vi "Laser Ablation and Capture.vi"() -> ()   [LabVIEW 2016] (continued)
          }
          frame True {
          }
        }
      }
    }
    n235 = call "uc480_SubVI_Example_SyncEventLoop.vi"("Error In"=w84, "use sync"=w86, ".NET (Reference)"=w85) -> ("Error Out"=w82:errorcluster, "Synchronize (ms)"=w83:dbl)  [unwired: 7 in]
    "Error Out" <- w82
    n236 = Wait Until Next ms Multiple(millisecond multiple=w83) -> ()  [unwired: 1 out]
  }
  n237 = flat-sequence "Initialization sequence" {
    tunnel: [w597] -> w38
    tunnel: [w581] -> w36
    tunnel: [w580] -> w35
    tunnel: [w577] -> w33
    tunnel: [w576] -> w32
    tunnel: [w573] -> w21
    tunnel: [w572] -> w2
    tunnel: [w571] -> w1
    tunnel: w38 -> [w739]
    tunnel: [w733] -> w37
    tunnel: w36 -> [w732]
    tunnel: w35 -> [w731]
    tunnel: [w730] -> w34
    tunnel: w33 -> [w730]
    tunnel: w32 -> [w729]
    tunnel: [w729] -> w31
    tunnel: [w728] -> w22
    tunnel: w21 -> [w728]
    tunnel: [w727] -> w10
    tunnel: [w726] -> w6
    tunnel: w2 -> [w727]
    tunnel: w1 -> [w726]
    tunnel: [w754] -> w49
    tunnel: [w745] -> w48
    tunnel: [w746] -> w44
    tunnel: w37 -> [w750]
    tunnel: w34 -> [w744]
    tunnel: w31 -> [w743]
    tunnel: [w742] -> w23
    tunnel: w22 -> [w742]
    tunnel: w10 -> [w741]
    tunnel: [w741] -> w9
    tunnel: w6 -> [w740]
    tunnel: [w740] -> w5
    tunnel: w49 -> [w760]
    tunnel: [w760] -> w47
    tunnel: w48 -> [w759]
    tunnel: [w758] -> w45
    tunnel: w44 -> [w758]
    tunnel: [w757] -> w30
    tunnel: w23 -> [w757]
    tunnel: w9 -> [w756]
    tunnel: [w756] -> w8
    tunnel: w5 -> [w755]
    tunnel: [w755] -> w4
    tunnel: w47 -> [w767]
    tunnel: [w767] -> w46
    tunnel: w45 -> [w766]
    tunnel: w30 -> [w765]
    tunnel: [w765] -> w29
    tunnel: w8 -> [w764]
    tunnel: [w764] -> w7
    tunnel: w4 -> [w763]
    tunnel: [w763] -> w3
    tunnel: [w777] -> w43
    tunnel: w46 -> [w777]
    tunnel: w29 -> [w772]
    tunnel: [w772] -> w28
    tunnel: [w771] -> w20
    tunnel: [w770] -> w15
    tunnel: w7 -> [w771]
    tunnel: w3 -> [w770]
    tunnel: w43 -> [w782]
    tunnel: [w782] -> w42
    tunnel: w28 -> [w780]
    tunnel: [w780] -> w27
    tunnel: w20 -> [w779]
    tunnel: [w779] -> w19
    tunnel: w15 -> [w778]
    tunnel: [w778] -> w14
    tunnel: w42 -> [w787]
    tunnel: [w787] -> w41
    tunnel: w27 -> [w785]
    tunnel: [w785] -> w26
    tunnel: w19 -> [w784]
    tunnel: [w784] -> w18
    tunnel: w14 -> [w783]
    tunnel: [w783] -> w13
    tunnel: w41 -> [w792]
    tunnel: [w792] -> w40
    tunnel: w26 -> [w790]
    tunnel: [w790] -> w25
    tunnel: w18 -> [w789]
    tunnel: [w789] -> w17
    tunnel: w13 -> [w788]
    tunnel: [w788] -> w12
    tunnel: w40 -> [w797]
    tunnel: [w797] -> w39
    tunnel: w25 -> [w795]
    tunnel: [w795] -> w24
    tunnel: w17 -> [w794]
    tunnel: [w794] -> w16
    tunnel: w12 -> [w793]
    tunnel: [w793] -> w11
    tunnel: w39 -> [w801]
    tunnel: w24 -> [w800]
    tunnel: w16 -> [w799]
    tunnel: w11 -> [w798]
    frame #0 {
      w598 = "standby" ("regular expression")
      w608 = FALSE ("Visible")
      n238 = control-ref of="This VI"() -> (w609:refnum<vi>)
      n239 = control-ref of="This VI"() -> (w607:refnum<vi>)
      n240 = invoke class="VI" method="Default Vals.Reinit All"(reference=w609) -> ()  [unwired: 2 in, 3 out]
      n241 = property on="Axes Manual Control" class="Bool (strict)"("Visible"=w608) -> ()  [unwired: 2 in, 2 out]
      n242 = property on="Home Axes" class="Bool"("Visible"=w608) -> ()  [unwired: 2 in, 2 out]
      n243 = property class="VI"(reference=w607) -> ("Path"=w606:path)  [unwired: 1 in, 2 out]
      n244 = Strip Path(path=w606) -> (stripped path=w605:path)  [unwired: 1 out]
      n245 = Build Path(base path=w605, name or relative path="General_Configuration.ini") -> (appended path=w603:path)
      n246 = call <vilib>:"Open Config Data.vi"("create file if necessary (T)"=FALSE, "configuration file path"=w603) -> ("error out"=w578:errorcluster, "refnum"=w579:T5)  [unwired: 7 in, 1 out]
      n247 = call "Configuration reader.vi"("refnum"=w579, "error in (no error)"=w578) -> ("Velocity"=→"Velocity":dbl, "Exposure"=w572:dbl, "X offset"=w590:i32, "Y travel"=w588:dbl, "X travel"=w587:dbl, "Y offset"=w589:i32, "Acceleration"=→"Acceleration":dbl, "Pixelclock"=w573:i32, "Framerate"=w571:dbl, "Width (px)"=w592:i32, "Speed (µm/s)"=w596:i32, "XPS_Address"=→"XPS_Address":string, "Axis 1 group"=w577:i32, "Precision (%)"=w593:dbl, "Pixel size"=w594:dbl, "Axis 2 inverted?"=→"Axis 2 inverted?":bool, "Axis 1 inverted?"=→"Axis 1 inverted?":bool, "Heigth (px)"=w591:i32, "Laser Com Delay"=w580:i32, "Height  step \ndivider"=w595:i32, "VISA Laser port"=w581:string, "Axis 2 group"=w576:i32, "error out"=w583:errorcluster)  [unwired: 3 in]
      "VISA Laser port" <- w581
      "Laser Com Delay" <- w580
      "Axis 1 group" <- w577
      "Axis 2 group" <- w576
      n248 = local write "Heigth (px)"(w591) -> ()
      n249 = local write "Pixel size"(w594) -> ()
      n250 = local write "Precision (%)"(w593) -> ()
      n251 = local write "Speed (µm/s)"(w596) -> ()
      n252 = local write "Width (px)"(w592) -> ()
      n253 = local write "Y offset"(w590) -> ()
      n254 = local write "X travel"(w587) -> ()
      n255 = local write "X offset"(w589) -> ()
      n256 = local write "Y travel"(w588) -> ()
      n257 = local write "Height \nstep divider"(w595) -> ()
      n258 = call "CheckStatus.vi"("Error In"=w583, "delay before read (ms)"=w580, "VISA resource name"=w581) -> ("Error Out"=w582:errorcluster, "read buffer"=w601:string)  [unwired: 5 in, 2 out]
      n259 = xnode "Match Regular Expression"("input string"=w601, "regular expression"=w598, "error in"=w582) -> ("whole match"=w599:string, "error out"=w597:errorcluster)  [unwired: 3 in, 3 out]
      n260 = Equal?(x=w599, y=w598) -> (x = y?=w600:bool)
      n261 = case shown="True" w600 {
        frame False {
        }
        frame True {
          n262 = control-ref of="Log"() -> (w725:refnum<vi>)
          n263 = call "Log writer.vi"("reference"=w725, "string"="Initializing the ICE450 Ultra..." ("Initialiazation")) -> ()  [unwired: 10 in]
        }
      }
    }
    frame #1 {
      n264 = call "ICE450 Ultra Initialization.vi"("error in (no error)"=w739, "delay before read (ms)"=w731, "VISA resource name"=w732) -> ("Error Out"=w733:errorcluster, "Repetition rate"=w734:dbl, "Laser initialization status"=w738:string)  [unwired: 6 in]
      n265 = local write "Repetition\nRate (Hz)"(w734) -> ()
      n266 = property on="Log" class="Str"("Text.Scroll Position"=u32 500000) -> ()  [unwired: 2 in, 2 out]
      n267 = Concatenate Strings(w738, "\r") -> (w736:string)
      n268 = invoke on="Log" class="Str" method="Append String"("string"=w736) -> ()  [unwired: 3 in, 4 out]
    }
    frame #2 {
      n269 = local read "XPS_Address"() -> (w747:string)
      n270 = control-ref of="Log"() -> (w748:refnum<vi>)
      n271 = call "Axes initialization.vi"("Axis 2 group"=w743, "Axis 1 group"=w744, "error in (no error)"=w750, "Axis Initial Parameters"="Axis Initial Parameters", "reference"=w748, "XPS_Address"=w747) -> ("Error out"=w751:errorcluster, "Axis 1"=→"Axis 1":string, "Axis 1 ready?"=w745:bool, "Axis 2"=→"Axis 2":string, "Axes 2 ready?"=w746:bool)
      n272 = call <vilib>:"Simple Error Handler.vi"("error in (no error)"=w751) -> ()  [unwired: 4 in, 5 out]
      n273 = And(x=w745, y=w746) -> (x .and. y?=w754:bool)
    }
    frame #3 {
      n274 = case shown="True" w759 {
        frame False {
        }
        frame True {
          n275 = control-ref of="Log"() -> (w762:refnum<vi>)
          n276 = call "Log writer.vi"("reference"=w762, "string"="Axis 1 ready" ("Initialiazation")) -> ()  [unwired: 10 in]
        }
      }
    }
    frame #4 {
      n277 = case shown="True" w766 {
        frame False {
        }
        frame True {
          n278 = control-ref of="Log"() -> (w768:refnum<vi>)
          n279 = call "Log writer.vi"("reference"=w768, "string"="Axis 2 ready" ("Initialiazation")) -> ()  [unwired: 10 in]
        }
      }
    }
    frame #5 {
      w773 = FALSE ("Visible")
      # "Set defaults"
      n280 = property on="LAMP" class="Bool (strict)"("BoolText.Text"="LAMP OFF" ("Boolean Text.Text")) -> ()  [unwired: 2 in, 2 out]
      n281 = property on="Laser Operation" class="Bool (strict)"("Blinking"=w773) -> ()  [unwired: 2 in, 2 out]
      n282 = property on="Capture" class="Bool"("Visible"=w773) -> ()  [unwired: 2 in, 2 out]
      n283 = property on="SINGLE SHOT" class="Bool"("Visible"=w773) -> ()  [unwired: 2 in, 2 out]
      n284 = property on="LASER" class="Bool (strict)"("BoolText.Text"="LASER OFF" ("Boolean Text.Text"), "Visible"=FALSE) -> ()  [unwired: 2 in, 2 out]
    }
    frame #6 {
      n285 = local write "Camera Status"("Init camera" ("Camera Status")) -> ()
    }
    frame #7 {
      n286 = Wait (ms)(milliseconds to wait=u32 1000) -> ()  [unwired: 1 out]
    }
    frame #8 {
      n287 = local write "Camera Status"("Start live") -> ()
    }
    frame #9 {
      n288 = Wait (ms)(milliseconds to wait=u32 1000) -> ()  [unwired: 1 out]
    }
    frame #10 {
      n289 = case shown="True" w801 {
        frame False {
          n290 = One Button Dialog(message="Axes not ready") -> ()  [unwired: 1 in, 1 out]
        }
        frame True {
          n291 = property on="Axes Manual Control" class="Bool (strict)"("Visible"=TRUE) -> ()  [unwired: 2 in, 2 out]
          n292 = property on="Home Axes" class="Bool"("Visible"=TRUE) -> ()  [unwired: 2 in, 2 out]
          n293 = control-ref of="Log"() -> (w804:refnum<vi>)
          n294 = call "Log writer.vi"("reference"=w804, "string"="System ready" ("Initialiazation")) -> ()  [unwired: 10 in]
        }
      }
      n295 = local write "Framerate"(w798) -> ()
      n296 = local write "Pixelclock"(w800) -> ()
      n297 = local write "Exposure"(w799) -> ()
    }
  }
  n298 = while "Laser control & Stages Control" {
    stop <- w819 stop-if-true
    n299 = local read "Laser Com Delay"() -> (w807:i32)
    n300 = local read "VISA Laser port"() -> (w808:string)
    n301 = local read "XPS_Address"() -> (w811:string)
    n302 = local read "Axis 2"() -> (w809:string)
    n303 = local read "Axis 1"() -> (w810:string)
    n304 = event shown="[12] \"Process Image\": Value Change" {
      selector: _ -> [_ _ _ _ _ _ _ _ _ _ _ _ _ _ _ _ _ _ _ _ _]
      dyn-events: _ -> [_ _ _ _ _ _ _ _ _ _ _ _ _ _ _ _ _ _ _ _ _]
      timeout: _ -> [_ _ _ _ _ _ _ _ _ _ _ _ _ _ _ _ _ _ _ _ _]
      tunnel: [_ _ _ w1151 _ _ _ _ _ _ _ _ _ _ _ _ _ _ _ _ _] -> w819
      tunnel: [w826 w982 w1145 _ _ _ _ w1212 _ w1240 w1267 _ w1331 _ _ _ "" ("StringOut") w1586 _ w1710 w1863] -> w812
      tunnel: w811 -> [_ _ _ _ _ _ _ _ _ _ w1270 _ _ _ _ _ w1503 w1585 _ w1697 w1854]
      tunnel: w810 -> [_ _ _ _ _ _ _ _ _ _ w1269 _ _ _ _ _ w1502 w1584 _ w1696 w1864]
      tunnel: w809 -> [_ _ _ _ _ _ _ _ _ _ w1268 _ _ _ _ _ w1501 w1583 _ w1695 w1865]
      tunnel: w808 -> [w824 w980 w1142 w1150 _ _ _ w1215 w1235 _ _ _ _ _ _ _ _ _ _ _ _]
      tunnel: w807 -> [w823 w979 w1141 w1149 _ _ _ w1214 w1234 _ _ _ _ _ _ _ _ _ _ _ _]
      event "LAMP": Value Change {
        n305 = event-data() -> ()  [unwired: 1 in, 6 out]
        n306 = case shown="True" "LAMP" {
          tunnel: [w827 w955] -> w826
          tunnel: w824 -> [w833 w954]
          tunnel: w823 -> [w832 w953]
          frame False {
            w828 = "standby" ("regular expression")
            n307 = call "FLStop.vi"("delay before read (ms)"=w832, "VISA resource name"=w833) -> ("read buffer"=w831:string)  [unwired: 6 in, 3 out]
            n308 = xnode "Match Regular Expression"("input string"=w831, "regular expression"=w828) -> ("whole match"=w829:string)  [unwired: 4 in, 4 out]
            n309 = Equal?(x=w829, y=w828) -> (x = y?=w830:bool)
            n310 = case shown="True" w830 {
              tunnel: ["" "Flashlamp deactivated"] -> w827
              frame False {
              }
              frame True {
                w835 = FALSE ("Visible")
                n311 = property on="LASER" class="Bool (strict)"("Visible"=w835) -> ()  [unwired: 2 in, 2 out]
                n312 = property on="Capture" class="Bool"("Visible"=w835) -> ()  [unwired: 2 in, 2 out]
                n313 = property on="SINGLE SHOT" class="Bool"("Visible"=w835) -> ()  [unwired: 2 in, 2 out]
                n314 = property on="Laser Operation" class="Bool (strict)"("Blinking"=w835) -> ()  [unwired: 2 in, 2 out]
                n315 = property on="LAMP" class="Bool (strict)"("BoolText.Text"="LAMP OFF" ("Boolean Text.Text")) -> ()  [unwired: 2 in, 2 out]
              }
            }
          }
          frame True {
            n316 = flat-sequence {
              tunnel: w954 -> [w963]
              tunnel: w953 -> [w962]
              tunnel: [w959] -> w952
              tunnel: [w973] -> w955
              tunnel: w952 -> [w972]
              frame #0 {
                w960 = "fire" ("regular expression")
                n317 = while {
                  i -> [w967]
                  stop <- w970 stop-if-true
                  n318 = Wait Until Next ms Multiple(millisecond multiple=u32 1000) -> ()  [unwired: 1 out]
                  n319 = Equal?(x=5, y=w967) -> (x = y?=w970:bool)
                  n320 = Subtract(x=5, y=w967) -> (x-y=w965:i32)
                  n321 = Number To Decimal String(number=w965) -> (decimal integer string=w966:string)  [unwired: 1 in]
                  n322 = property on="LAMP" class="Bool (strict)"("BoolText.Text"=w966) -> ()  [unwired: 2 in, 2 out]
                }
                n323 = Wait (ms)(milliseconds to wait=u32 5000) -> ()  [unwired: 1 out]
                n324 = call "FLStart.vi"("delay before read (ms)"=w962, "VISA resource name"=w963) -> ("Error Out"=w957:errorcluster, "read buffer"=w958:string)  [unwired: 6 in, 2 out]
                n325 = Match Pattern(string=w958, regular expression=w960) -> (match substring=w961:string)  [unwired: 1 in, 3 out]
                n326 = call <vilib>:"Simple Error Handler.vi"("error source (\" \")"="Lamp" ("error source (\" \")"), "error in (no error)"=w957) -> ()  [unwired: 3 in, 5 out]
                n327 = Equal?(x=w961, y=w960) -> (x = y?=w959:bool)
              }
              frame #1 {
                n328 = case shown="True" w972 {
                  tunnel: ["Flashlamp NOT firing" "Flashlamp activated"] -> w973
                  frame False {
                    n329 = property on="LAMP" class="Bool (strict)"("Value"=FALSE ("LAMP")) -> ()  [unwired: 2 in, 2 out]
                  }
                  frame True {
                    w976 = TRUE ("Visible")
                    n330 = property on="LASER" class="Bool (strict)"("Visible"=w976) -> ()  [unwired: 2 in, 2 out]
                    n331 = property on="Capture" class="Bool"("Visible"=w976) -> ()  [unwired: 2 in, 2 out]
                    n332 = property on="LAMP" class="Bool (strict)"("BoolText.Text"="LAMP ON" ("Boolean Text.Text")) -> ()  [unwired: 2 in, 2 out]
                    n333 = property on="SINGLE SHOT" class="Bool"("Visible"=w976) -> ()  [unwired: 2 in, 2 out]
                  }
                }
              }
            }
          }
        }
      }
      event "LASER": Value Change {
        n334 = event-data() -> ()  [unwired: 1 in, 6 out]
        n335 = case shown="False" "LASER" {
          tunnel: [w993 w1122] -> w983
          tunnel: [w992 w1121] -> w982
          tunnel: w980 -> [w990 w1116]
          tunnel: w979 -> [w989 w1115]
          frame False {
            w987 = "fire" ("regular expression")
            n336 = local read "LAMP"() -> (w991:bool)
            n337 = case shown="True" w991 {
              tunnel: [FALSE ("Visible") TRUE ("Visible")] -> w984
              frame False {
              }
              frame True {
              }
            }
            n338 = property on="Capture" class="Bool"("Visible"=w984) -> ()  [unwired: 2 in, 2 out]
            n339 = property on="SINGLE SHOT" class="Bool"("Visible"=w984) -> ()  [unwired: 2 in, 2 out]
            n340 = call "QSStop.vi"("delay before read (ms)"=w989, "VISA resource name"=w990) -> ("read buffer"=w986:string)  [unwired: 6 in, 3 out]
            n341 = xnode "Match Regular Expression"("input string"=w986, "regular expression"=w987) -> ("whole match"=w988:string)  [unwired: 4 in, 4 out]
            n342 = Equal?(x=w988, y=w987) -> (x = y?=w985:bool)
            n343 = case shown="False" w985 {
              tunnel: [FALSE w997] -> w993
              tunnel: ["" "Q-Switch deactivated"] -> w992
              frame False {
              }
              frame True {
                w997 = FALSE ("Boolean")
                n344 = property on="LASER" class="Bool (strict)"("BoolText.Text"="LASER OFF" ("Boolean Text.Text"), "Value"=w997) -> ()  [unwired: 2 in, 2 out]
                n345 = property on="Laser Operation" class="Bool (strict)"("Blinking"=w997) -> ()  [unwired: 2 in, 2 out]
              }
            }
          }
          frame True {
            w1118 = "fire" ("regular expression")
            n346 = call "CheckStatus.vi"("delay before read (ms)"=w1115, "VISA resource name"=w1116) -> ("read buffer"=w1120:string)  [unwired: 6 in, 3 out]
            n347 = Match Pattern(string=w1120, regular expression=w1118) -> (match substring=w1119:string)  [unwired: 1 in, 3 out]
            n348 = Equal?(x=w1119, y=w1118) -> (x = y?=w1117:bool)
            n349 = case shown="True" w1117 {
              tunnel: [FALSE ("Boolean") w1133] -> w1122
              tunnel: ["The flashlamp is not firing" w1132] -> w1121
              tunnel: w1116 -> [_ w1131]
              tunnel: w1115 -> [_ w1130]
              frame False {
                n350 = property on="LASER" class="Bool (strict)"("Value"=FALSE ("LASER")) -> ()  [unwired: 2 in, 2 out]
              }
              frame True {
                w1128 = "qs" ("regular expression")
                n351 = call "QSStart.vi"("delay before read (ms)"=w1130, "VISA resource name"=w1131) -> ("read buffer"=w1127:string)  [unwired: 6 in, 3 out]
                n352 = Match Pattern(string=w1127, regular expression=w1128) -> (match substring=w1129:string)  [unwired: 1 in, 3 out]
                n353 = Equal?(x=w1129, y=w1128) -> (x = y?=w1126:bool)
                n354 = case shown="True" w1126 {
                  tunnel: [FALSE ("Boolean") w1139] -> w1133
                  tunnel: ["Q-Switch is NOT firing" "Q-Switch activated"] -> w1132
                  frame False {
                    n355 = property on="LASER" class="Bool (strict)"("Value"=FALSE ("LASER")) -> ()  [unwired: 2 in, 2 out]
                  }
                  frame True {
                    w1137 = FALSE ("Visible")
                    w1139 = TRUE ("Boolean")
                    n356 = property on="Capture" class="Bool"("Visible"=w1137) -> ()  [unwired: 2 in, 2 out]
                    n357 = property on="Laser Operation" class="Bool (strict)"("Blinking"=w1139) -> ()  [unwired: 2 in, 2 out]
                    n358 = property on="LASER" class="Bool (strict)"("BoolText.Text"="LASER ON" ("Boolean Text.Text")) -> ()  [unwired: 2 in, 2 out]
                    n359 = property on="SINGLE SHOT" class="Bool"("Visible"=w1137) -> ()  [unwired: 2 in, 2 out]
                  }
                }
              }
            }
          }
        }
        "Laser Operation" <- w983
      }
      event "Repetition\nRate (Hz)": Value Change {
        n360 = event-data() -> ()  [unwired: 1 in, 6 out]
        n361 = call "FLFrequencySet.vi"("Frequency (Hz)"="Repetition\nRate (Hz)", "delay before read (ms)"=w1141, "VISA resource name"=w1142) -> ()  [unwired: 5 in, 4 out]
        n362 = Number To Fractional String(number="Repetition\nRate (Hz)", precision (6)=i16 2 ("width (-)")) -> (F-format string=w1147:string)  [unwired: 2 in]
        n363 = Concatenate Strings("Repetition rate set to: " ("string"), w1147, " Hz" ("string")) -> (w1145:string)
      }
      event "EXIT": Value Change {
        n364 = event-data() -> ()  [unwired: 1 in, 6 out]
        n365 = flat-sequence {
          tunnel: w1150 -> [w1153]
          tunnel: w1149 -> [w1152]
          tunnel: ["EXIT"] -> w1151
          frame #0 {
            n366 = call "QSStop.vi"("delay before read (ms)"=w1152, "VISA resource name"=w1153) -> ("Error Out"=w1154:errorcluster)  [unwired: 6 in, 3 out]
            n367 = call "FLStop.vi"("Error In"=w1154, "delay before read (ms)"=w1152, "VISA resource name"=w1153) -> ()  [unwired: 5 in, 4 out]
          }
          frame #1 {
            n368 = Wait (ms)(milliseconds to wait=u32 1000) -> ()  [unwired: 1 out]
          }
          frame #2 {
            n369 = local write "Camera Status"("Exit camera") -> ()
          }
          frame #3 {
            n370 = Wait (ms)(milliseconds to wait=u32 1000) -> ()  [unwired: 1 out]
          }
          frame #4 {
            n371 = control-ref of="This Application"() -> (w1175:refnum<vi>)
            n372 = call "Personal document path.vi"() -> ("My Documents"=w1158:path)  [unwired: 10 in, 1 out]
            n373 = property class="App"(reference=w1175) -> ("App.Kind"=w1174:T8)  [unwired: 1 in, 2 out]
            n374 = Build Path(base path=w1158, name or relative path="Laser Ablation and Capture - Logs") -> (appended path=w1168:path)
            n375 = case shown="\"Run Time System\"" w1174 {
              frame "Development System", Default {
              }
              frame "Run Time System" {
                n376 = control-ref of="This VI"() -> (w1184:refnum<vi>)
                n377 = invoke class="VI" method="FP.Close"(reference=w1184) -> ()  [unwired: 2 in, 3 out]
                n378 = Quit LabVIEW() -> ()  [unwired: 1 in]
              }
            }
            n379 = call <vilib>:"Check if File or Folder Exists.vi"("path"=w1168) -> ("file or folder exists?"=w1169:bool, "dup path"=w1170:path)  [unwired: 8 in, 1 out]
            n380 = case shown="False" w1169 {
              tunnel: w1170 -> [w1177 w1178]
              tunnel: [w1176 w1178] -> w1173
              frame False {
                n381 = Create Folder(path (use dialog)=w1177) -> (created path=w1176:path)  [unwired: 2 in, 2 out]
              }
              frame True {
              }
            }
            n382 = Get Date/Time In Seconds() -> (seconds since 1Jan1904=w1166:timestamp)
            n383 = Format Date/Time String(time format string (%c)="%d%m%y %I-%M %p ", seconds (now)=w1166) -> (date/time string=w1164:string)  [unwired: 1 in]
            n384 = Concatenate Strings(w1164, "Log File.txt") -> (w1172:string)
            n385 = Build Path(base path=w1173, name or relative path=w1172) -> (appended path=w1171:path)
            n386 = Open/Create/Replace File(file path (use dialog)=w1171, operation (0:open)=T6."replace or create") -> (refnum out=w1162:refnum<file>, cancelled=w1160:bool, error out=w1161:errorcluster)  [unwired: 4 in]
            n387 = case shown="False" w1160 {
              tunnel: w1162 -> [w1183 _]
              tunnel: w1161 -> [w1181 _]
              frame False {
                n388 = local read "Log"() -> (w1182:string)
                n389 = Write to Text File(file (use dialog)=w1183, text=w1182, error in=w1181) -> (refnum out=w1180:refnum<file>, error out=w1179:errorcluster)  [unwired: 2 out]
                n390 = Close File(refnum=w1180, error in=w1179) -> ()  [unwired: 2 out]
              }
              frame True {
              }
            }
          }
          frame #5 {
          }
        }
      }
      event "Log files": Value Change {
        n391 = event-data() -> ()  [unwired: 1 in, 6 out]
        n392 = case shown="True" "Log files" {
          frame False {
          }
          frame True {
            n393 = call "Personal document path.vi"() -> ("My Documents"=w1188:path)  [unwired: 10 in, 1 out]
            n394 = Build Path(base path=w1188, name or relative path="Laser Ablation and Capture - Logs") -> (appended path=w1187:path)
            n395 = Path To String(path=w1187) -> (string=w1193:string)
            n396 = Concatenate Strings("cmd /c explorer.exe " ("string"), w1193) -> (w1191:string)
            n397 = call <vilib>:"System Exec.vi"("run minimized? (F)"=TRUE, "command line"=w1191) -> ()  [unwired: 6 in, 4 out]
          }
        }
      }
      event "Processing time unit", "Processi time (sec)": Value Change {
        n398 = event-data() -> ()  [unwired: 1 in, 6 out]
        n399 = local read "Processing time unit"() -> (w1196:string)
        n400 = Equal?(x=w1196, y="min") -> (x = y?=w1194:bool)
        n401 = case shown="False" w1194 {
          frame False {
            n402 = local read "Processi time (sec)"() -> (w1197:i32)
            n403 = local write "Process time"(w1197) -> ()
          }
          frame True {
            n404 = local read "Processi time (sec)"() -> (w1199:i32)
            n405 = Quotient & Remainder(x=w1199, y=60) -> (floor(x/y)=w1198:i32)  [unwired: 1 out]
            n406 = local write "Process time"(w1198) -> ()
          }
        }
      }
      event "Overlay MSI Image": Value Change {
        n407 = event-data() -> ()  [unwired: 1 in, 6 out]
        n408 = vi-ref "MSI_Image_overlap.vi"() -> (w1201:refnum<vi>)
        n409 = case shown="True" "Overlay MSI Image" {
          tunnel: w1201 -> [_ w1206]
          frame False {
          }
          frame True {
            n410 = invoke class="VI" method="FP.Open"(reference=w1206, "Activate"=TRUE ("Activate?"), "State"=T7."Standard") -> (reference out=w1209:refnum<vi>, error out=w1204:errorcluster)  [unwired: 2 in, 3 out]
            n411 = invoke class="VI" method="Run VI"(reference=w1209, error in=w1204, "Wait until done"=FALSE ("Wait Until Done"), "Auto Dispose Ref"=TRUE ("Auto Dispose Reference")) -> (reference out=w1205:refnum<vi>, error out=w1203:errorcluster)  [unwired: 1 in, 3 out]
            n412 = Close Reference(reference=w1205, error in (no error)=w1203) -> ()  [unwired: 1 out]
          }
        }
      }
      event "SINGLE SHOT": Value Change {
        n413 = event-data() -> ()  [unwired: 1 in, 6 out]
        n414 = case shown="True" "SINGLE SHOT" {
          tunnel: w1215 -> [_ w1219]
          tunnel: w1214 -> [_ w1218]
          tunnel: ["" w1217] -> w1212
          frame False {
          }
          frame True {
            w1223 = "fire" ("regular expression")
            n415 = call "CheckStatus.vi"("delay before read (ms)"=w1218, "VISA resource name"=w1219) -> ("read buffer"=w1221:string)  [unwired: 6 in, 3 out]
            n416 = Match Pattern(string=w1221, regular expression=w1223) -> (match substring=w1222:string)  [unwired: 1 in, 3 out]
            n417 = Equal?(x=w1222, y=w1223) -> (x = y?=w1220:bool)
            n418 = case shown="True" w1220 {
              tunnel: ["The flashlamp is not firing" w1231] -> w1217
              tunnel: w1219 -> [_ w1230]
              tunnel: w1218 -> [_ w1229]
              frame False {
              }
              frame True {
                w1227 = "qs" ("regular expression")
                n419 = call "QSSingleShot.vi"("delay before read (ms)"=w1229, "VISA resource name"=w1230) -> ("read buffer"=w1226:string)  [unwired: 6 in, 3 out]
                n420 = Match Pattern(string=w1226, regular expression=w1227) -> (match substring=w1228:string)  [unwired: 1 in, 3 out]
                n421 = Equal?(x=w1228, y=w1227) -> (x = y?=w1225:bool)
                n422 = case shown="True" w1225 {
                  tunnel: ["Q-Switch is NOT firing" "Q-Switch activated"] -> w1231
                  frame False {
                  }
                  frame True {
                  }
                }
              }
            }
          }
        }
      }
      event "Laser Status": Value Change {
        n423 = event-data() -> ()  [unwired: 1 in, 6 out]
        n424 = case shown="True" "Laser Status" {
          tunnel: w1235 -> [_ w1238]
          tunnel: w1234 -> [_ w1237]
          frame False {
          }
          frame True {
            n425 = call "ICE450UltraMonitor.vi"("delay before read (ms)"=w1237, "VISA resource name"=w1238) -> ()  [unwired: 10 in]
          }
        }
      }
      event "Open \nManual": Value Change {
        n426 = event-data() -> ()  [unwired: 1 in, 6 out]
        n427 = case shown="True" "Open \nManual" {
          tunnel: [_ "Opening Manual" ("StringOut")] -> w1240
          frame False {
          }
          frame True {
            w1249 = FALSE  # wait until completion? (T)
            n428 = control-ref of="This VI"() -> (w1253:refnum<vi>)
            n429 = property class="VI"(reference=w1253) -> ("Path"=w1252:path)  [unwired: 1 in, 2 out]
            n430 = Strip Path(path=w1252) -> (stripped path=w1251:path)  [unwired: 1 out]
            n431 = Build Path(base path=w1251, name or relative path="LAST_Software_Manual.PDF") -> (appended path=w1243:path)
            n432 = Path To String(path=w1243) -> (string=w1246:string)
            n433 = Concatenate Strings("cmd  /c \"", w1246, "\"" ("string")) -> (w1241:string)
            n434 = call <vilib>:"System Exec.vi"("run minimized? (F)"=TRUE, "wait until completion? (T)"=w1249, "error in (no error)"="error in (no error)", "command line"=w1241) -> ("error out"=→"error out":errorcluster)  [unwired: 4 in, 3 out]
          }
        }
      }
      event "Stages status": Value Change {
        w1261 = "Ready"
        n435 = event-data() -> ()  [unwired: 1 in, 6 out]
        n436 = case shown="True" "Stages status" {
          tunnel: w1270 -> [_ w1283]
          tunnel: w1269 -> [_ w1282]
          tunnel: w1268 -> [_ w1281]
          tunnel: [w1274 w1280] -> w1267
          tunnel: [w1274 w1278] -> w1257
          tunnel: [w1274 w1279] -> w1256
          frame False {
            w1274 = ""
          }
          frame True {
            n437 = call <userlib>:"Open TCP-IP.vi"("IP address"=w1283) -> ("error out"=w1277:errorcluster, "Connection ID"=w1284:T9)  [unwired: 8 in, 1 out]
            n438 = call <vilib>:"Simple Error Handler.vi"("error in (no error)"=w1277) -> ("error?"=w1275:bool, "error out"=w1276:errorcluster)  [unwired: 4 in, 3 out]
            n439 = case shown="False" w1275 {
              tunnel: w1284 -> [w1305 _]
              tunnel: w1276 -> [w1304 _]
              tunnel: w1282 -> [w1297 _]
              tunnel: w1281 -> [w1296 _]
              tunnel: [w1295 w1306] -> w1280
              tunnel: [w1292 w1306] -> w1279
              tunnel: [w1288 w1306] -> w1278
              frame False {
                n440 = call "Get Stages Status.vi"("error in (no error)"=w1304, "Group Name (250 c max)"=w1297, "connection ID in"=w1305) -> ("error out"=w1301:errorcluster, "XPS error out"=w1300:errorcluster, "Group Status String"=w1292:string, "connection ID out"=w1303:T9)  [unwired: 4 in, 1 out]
                n441 = call "Get Stages Status.vi"("error in (no error)"=w1301, "XPS error in (no error)"=w1300, "Group Name (250 c max)"=w1296, "connection ID in"=w1303) -> ("error out"=w1298:errorcluster, "XPS error out"=w1294:errorcluster, "Group Status String"=w1288:string, "connection ID out"=w1299:T9)  [unwired: 3 in, 1 out]
                n442 = call <vilib>:"Simple Error Handler.vi"("error source (\" \")"="Stage status" ("error source (\" \")"), "error in (no error)"=w1294) -> ()  [unwired: 3 in, 5 out]
                n443 = Concatenate Strings("Axis 1 " ("string"), w1292) -> (w1291:string)
                n444 = call <userlib>:"Close TCP-IP.vi"("error in (no error)"=w1298, "connection ID in"=w1299) -> ("Error out"=w1293:errorcluster)  [unwired: 9 in]
                n445 = call <vilib>:"Simple Error Handler.vi"("error source (\" \")"="TCP close Stage status" ("error source (\" \")"), "error in (no error)"=w1293) -> ()  [unwired: 3 in, 5 out]
                n446 = Concatenate Strings("Axis 2 " ("string"), w1288) -> (w1289:string)
                n447 = Concatenate Strings(w1291, " - " ("string"), w1289) -> (w1295:string)
              }
              frame True {
                w1306 = ""
              }
            }
          }
        }
        n448 = String Subset(string=w1256, offset (0)=0, length (rest)=5 ("length (rest)")) -> (substring=w1260:string)
        n449 = String Subset(string=w1257, offset (0)=0, length (rest)=5 ("length (rest)")) -> (substring=w1262:string)
        n450 = Equal?(x=w1261, y=w1260) -> (x = y?=w1258:bool)
        n451 = Equal?(x=w1262, y=w1261) -> (x = y?=w1259:bool)
        n452 = And(x=w1259, y=w1258) -> (x .and. y?=w1255:bool)
        n453 = case shown="True" w1255 {
          frame False {
          }
          frame True {
            n454 = property on="Axes Manual Control" class="Bool (strict)"("Visible"=TRUE) -> ()  [unwired: 2 in, 2 out]
            n455 = property on="Home Axes" class="Bool"("Visible"=TRUE) -> ()  [unwired: 2 in, 2 out]
          }
        }
      }
      event "Save configuration": Value Change {
        n456 = event-data() -> ()  [unwired: 1 in, 6 out]
        n457 = case shown="True" "Save configuration" {
          frame False {
          }
          frame True {
            n458 = control-ref of="This VI"() -> (w1329:refnum<vi>)
            n459 = local read "Pixelclock"() -> (w1310:i32)
            n460 = local read "Framerate"() -> (w1309:dbl)
            n461 = local read "Exposure"() -> (w1308:dbl)
            n462 = property class="VI"(reference=w1329) -> ("Path"=w1328:path)  [unwired: 1 in, 2 out]
            n463 = Strip Path(path=w1328) -> (stripped path=w1327:path)  [unwired: 1 out]
            n464 = local read "Height \nstep divider"() -> (w1322:i32)
            n465 = Build Path(base path=w1327, name or relative path="General_Configuration.ini") -> (appended path=w1325:path)
            n466 = local read "Speed (µm/s)"() -> (w1318:i32)
            n467 = local read "Precision (%)"() -> (w1319:dbl)
            n468 = local read "Heigth (px)"() -> (w1321:i32)
            n469 = local read "Width (px)"() -> (w1317:i32)
            n470 = local read "Pixel size"() -> (w1320:dbl)
            n471 = local read "Y offset"() -> (w1316:i32)
            n472 = local read "X travel"() -> (w1314:dbl)
            n473 = local read "X offset"() -> (w1315:i32)
            n474 = local read "Y travel"() -> (w1313:dbl)
            n475 = call <vilib>:"Open Config Data.vi"("create file if necessary (T)"=FALSE, "configuration file path"=w1325) -> ("error out"=w1312:errorcluster, "refnum"=w1323:T5)  [unwired: 7 in, 1 out]
            n476 = call "Configuration writer.vi"("Path"=w1323, "Width (px)"=w1317, "error in (no error)"=w1312, "Precision (%)"=w1319, "Heigth (px)"=w1321, "X offset"=w1316, "X travel"=w1314, "Y offset"=w1315, "Speed (µm/s)"=w1318, "Height  step \ndivider"=w1322, "Y travel"=w1313, "Pixel size"=w1320, "Pixelclock"=w1310, "Framerate"=w1309, "Exposure"=w1308) -> ("error out"=w1311:errorcluster)  [unwired: 4 in]
            n477 = call <vilib>:"Simple Error Handler.vi"("error in (no error)"=w1311) -> ()  [unwired: 4 in, 5 out]
          }
        }
      }
      event "Process Image": Value Change {
        n478 = event-data() -> ()  [unwired: 1 in, 6 out]
        n479 = case shown="True" "Process Image" {
          tunnel: ["" "Processing done"] -> w1331
          frame False {
          }
          frame True {
            w1360 = 0.2  # Delay after laser on/off
            w1420 = i16 6 ("precision (6)")
            w1416 = 1000 ("y")
            n480 = local read "Width (px)"() -> (w1378:i32)
            n481 = local read "Source"() -> (w1419:T2)
            n482 = control-ref of="This VI"() -> (w1344:refnum<vi>)
            n483 = control-ref of="This VI"() -> (w1336:refnum<vi>)
            n484 = property on="Source" class="ImageControl"() -> ("ROI"=w1335:T10)  [unwired: 2 in, 2 out]
            n485 = property class="VI"(reference=w1344) -> ("Path"=w1343:path)  [unwired: 1 in, 2 out]
            n486 = property class="VI"(reference=w1336) -> ("Path"=w1337:path)  [unwired: 1 in, 2 out]
            n487 = call "ROI preparation.vi"("ROI"=w1335, "Width (px)"=w1378, "Refnum in"=w1419) -> ("error out"=w1392:errorcluster, "ROI Empty?"=w1374:bool, "Global Rectangle[0]\nX"=w1355:i32, "Corrected ROI"=w1375:u8[][], "Global Rectangle[1]\nY"=w1356:i32, "Rect width \n(px)"=w1334:i32, "Rect height \n(px)"=w1333:i32)  [unwired: 1 in, 1 out]
            "Rect width\n(px)" <- w1334
            "Rect height\n(px)" <- w1333
            n488 = Divide(x=w1378, y=2) -> (x/y=w1382:dbl)
            n489 = local read "Y offset"() -> (w1386:i32)
            n490 = local read "X offset"() -> (w1387:i32)
            n491 = call <vilib>:"Simple Error Handler.vi"("error in (no error)"=w1392) -> ()  [unwired: 4 in, 5 out]
            n492 = Strip Path(path=w1343) -> (stripped path=w1342:path)  [unwired: 1 out]
            n493 = Strip Path(path=w1337) -> (stripped path=w1338:path)  [unwired: 1 out]
            n494 = Round To Nearest(number=w1382) -> (nearest integer value=w1373:dbl)
            n495 = Initialize Array(1 ("element"), w1378, w1378) -> (w1383:i32[][])
            n496 = case shown="True" w1374 {
              tunnel: [w1431 u8[][] [[1]] ("Image Pixels (U8)")] -> w1409
              tunnel: w1375 -> [w1431 _]
              frame False {
              }
              frame True {
                n497 = One Button Dialog(message="ATTENTION: you did not select\nany region of interest") -> ()  [unwired: 1 in, 1 out]
              }
            }
            n498 = call "Circle Spot Calculator.vi"("Center Y"=w1373, "Radius"=w1373, "Center X"=w1373, "initialized array"=w1383) -> ("Array"=w1380:i32[][])  [unwired: 6 in]
            n499 = Subtract(x=w1356, y=w1386) -> (x-y=w1376:i32)
            n500 = Subtract(x=w1355, y=w1387) -> (x-y=w1377:i32)
            n501 = Add Array Elements(numeric array=w1380) -> (sum=w1379:i32)
            n502 = Build Path(base path=w1342, name or relative path="Last_ROI.TIFF") -> ()  [unwired: 1 out]
            n503 = Build Path(base path=w1338, name or relative path="Last_ROI.TIFF") -> (appended path=w1340:path)
            n504 = call "Save ROI.vi"("File path"=w1340, "ROI"=w1335) -> ()  [unwired: 10 in]
            n505 = local read "Height \nstep divider"() -> (w1370:i32)
            n506 = local read "Heigth (px)"() -> (w1371:i32)
            n507 = local read "Pixel size"() -> (w1388:dbl)
            n508 = Divide "Height of a line"(x=w1371, y=w1370) -> (x/y=w1394:dbl)
            n509 = Multiply(x=w1333, y=w1388) -> (x*y=w1402:dbl)
            n510 = Multiply(x=w1388, y=w1376) -> (x*y=w1390:dbl)
            n511 = Multiply(x=w1377, y=w1388) -> (x*y=w1389:dbl)
            n512 = Multiply(x=w1334, y=w1388) -> (x*y=w1403:dbl)
            n513 = Multiply(x=w1388, y=w1388) -> (x*y=w1412:dbl)
            n514 = To Double Precision Float(number=w1409) -> (double precision float=w1410:dbl[][])
            n515 = call "ROI parser.vi"("Circle spot"=w1379, "Circle?"="Circle?", "ROI (8 bit image)"=w1409, "Ablation spot width"=w1378, "Sampling\nPrecision"="Precision (%)", "Ablation spot heigth"=w1371, "Height  step \ndivider"=w1370) -> ("Parsed array"=w1424:bool[][])  [unwired: 4 in]
            n516 = Add Array Elements(numeric array=w1410) -> (sum=w1414:dbl)
            n517 = Divide(x=w1390, y=w1416) -> (x/y=w1418:dbl)
            n518 = Divide(x=w1389, y=w1416) -> (x/y=w1417:dbl)
            n519 = Multiply(x=w1388, y=w1394) -> (x*y=w1395:dbl)
            n520 = Round To Nearest(number=w1402) -> (nearest integer value=→"Rect height\n(µm/px)":dbl)
            n521 = Round To Nearest(number=w1403) -> (nearest integer value=→"Rect. width \n(µm/px))":dbl)
            n522 = call "Array processor.vi"("Source array"=w1424, "Pixel size"=w1388) -> ("Lenght array"=w1391:dbl[][], "T/F product array"=w1398:bool[][])  [unwired: 8 in]
            n523 = Round To Nearest(number=w1395) -> (nearest integer value=w1393:dbl)
            n524 = Number To Fractional String(number=w1418, precision (6)=w1420) -> (F-format string=w1407:string)  [unwired: 2 in]
            n525 = Number To Fractional String(number=w1417, precision (6)=w1420) -> (F-format string=w1408:string)  [unwired: 2 in]
            n526 = Divide(x=w1414, y=u8 255) -> (x/y=w1411:dbl)
            n527 = local read "Axis 1 inverted?"() -> (w1365:bool)
            n528 = local read "Axis 2 inverted?"() -> (w1364:bool)
            n529 = local read "Speed (µm/s)"() -> (w1399:i32)
            n530 = Multiply(x=w1411, y=w1412) -> (x*y=w1406:dbl)
            n531 = Fract/Exp String To Number(string=w1407) -> (number=w1369:dbl)  [unwired: 3 in, 1 out]
            n532 = Fract/Exp String To Number(string=w1408) -> (number=w1368:dbl)  [unwired: 3 in, 1 out]
            n533 = Index Array(array=w1398, index (col)=0 ("disabled index (col)")) -> (element=w1422:bool[])  [unwired: 1 in]
            n534 = local read "Axis 1"() -> (w1401:string)
            n535 = local read "Axis 2"() -> (w1400:string)
            n536 = case shown="True" w1365 {
              tunnel: w1369 -> [w1428 w1430]
              tunnel: [w1428 w1429] -> w1367
              frame False {
              }
              frame True {
                n537 = Negate(x=w1430) -> (-x=w1429:dbl)
              }
            }
            "Axis 1 Offset" <- w1367
            n538 = case shown="True" w1364 {
              tunnel: w1368 -> [w1425 w1427]
              tunnel: [w1425 w1426] -> w1366
              frame False {
              }
              frame True {
                n539 = Negate(x=w1427) -> (-x=w1426:dbl)
              }
            }
            "Axis 2 Offset" <- w1366
            n540 = call "Commands array generator.vi"("Axis 1"=w1401, "Axis 1 inverted?"=w1365, "Axis in"=w1400, "Axis 2 inverted?"=w1364, "Axes speed \n(µm/s)"=w1399, "Y Step size in µm"=w1393, "T/F product array"=w1398, "Space defined array"=w1391) -> ("Command Array"=w1354:string[][], "Time Array"=w1359:dbl[][])  [unwired: 2 in]
            "Commands array" <- w1354
            n541 = Array Size(array=w1422) -> (size(s)=w1421:i32)
            n542 = for {
              N: w1421 -> [_]
              tunnel: w1398 -> [w1436] mode=indexing
              tunnel: [w1434] -> w1363 mode=indexing
              # "This loop add a F for each Y moviment"
              n543 = Build Array (concatenate)(w1436, FALSE) -> (w1434:bool[])
            }
            "Laser on/off array" <- w1363
            n544 = Divide(x=w1406, y=1000000.0) -> (x/y=→"ROI Area \n(mm2)":dbl)
            n545 = Add Array Elements(numeric array=w1359) -> (sum=w1357:dbl)
            n546 = Array Size(array=w1354) -> (size(s)=w1353:i32[])
            n547 = Array To Cluster(array=w1353) -> (cluster=w1352:cluster{"[0]":i32, "[1]":i32})
            n548 = Unbundle(w1352) -> ("[0]"=w1351:i32, "[1]"=w1350:i32)
            n549 = Multiply(x=w1351, y=w1350) -> (x*y=w1348:i32)
            n550 = Multiply(x="Captur time\nConstant", y=w1348) -> (x*y=w1347:dbl)
            n551 = Boolean To (0,1)(Boolean=w1363) -> (0, 1=w1362:i16[][])
            n552 = Add Array Elements(numeric array=w1362) -> (sum=w1361:i16)
            n553 = Multiply(x=w1360, y=w1361) -> (x*y=w1358:dbl)
            n554 = Add(x=w1358, y=w1357) -> (x+y=w1346:dbl)
            n555 = Add(x=w1346, y=w1347) -> (x+y=w1345:dbl)
            "Processi time (sec)" <- w1345
            n556 = local write "Process time"(w1345) -> ()
          }
        }
      }
      event "Call Last ROI": Value Change {
        n557 = event-data() -> ()  [unwired: 1 in, 6 out]
        n558 = control-ref of="This VI"() -> (w1437:refnum<vi>)
        n559 = property class="VI"(reference=w1437) -> ("Path"=w1440:path)  [unwired: 1 in, 2 out]
        n560 = Strip Path(path=w1440) -> (stripped path=w1439:path)  [unwired: 1 out]
        n561 = Build Path(base path=w1439, name or relative path="Last_ROI.TIFF") -> (appended path=w1443:path)
        n562 = call <vilib>:"Check if File or Folder Exists.vi"("path"=w1443) -> ("file or folder exists?"=w1442:bool)  [unwired: 8 in, 2 out]
        n563 = And(x=w1442, y="Call Last ROI") -> (x .and. y?=w1444:bool)
        n564 = case shown="True" w1444 {
          tunnel: w1443 -> [_ w1452]
          frame False {
          }
          frame True {
            n565 = call "IMAQ Create"("Image Name"="untitled") -> ("New Image"=w1454:T2)  [unwired: 4 in, 1 out]
            n566 = call "IMAQ ReadFile"("File Path"=w1452, "Image"=w1454) -> ("Image Out"=w1453:T2)  [unwired: 5 in, 4 out]
            n567 = call "IMAQ MaskToROI"("Image"=w1453) -> ("ROI Descriptor"=w1445:T11)  [unwired: 6 in, 2 out]
            n568 = Unbundle By Name(w1445) -> ("Contours"=w1450:T12)  [unwired: 1 out]
            n569 = Index Array(array=w1450) -> (element=w1451:T13)  [unwired: 1 in]
            n570 = Bundle By Name(cluster=w1451, "Type"=u32 6) -> (w1449:T13)
            n571 = Replace Array Subset(array=w1450, new element=w1449) -> (w1448:T12)  [unwired: 1 in]
            n572 = Bundle By Name(cluster=w1445, "Contours"=w1448) -> (w1446:T11)
            n573 = property on="Source" class="ImageControl"("ROI"=w1446) -> ()  [unwired: 2 in, 2 out]
          }
        }
      }
      event "Save current ROI": Value Change {
        n574 = event-data() -> ()  [unwired: 1 in, 6 out]
        n575 = property on="Source" class="ImageControl"() -> ("ROI"=w1461:T10)  [unwired: 2 in, 2 out]
        n576 = Unbundle By Name(w1461) -> ("Contours"=w1456:T14)
        n577 = Index Array(array=w1456) -> (element=w1457:T15)  [unwired: 1 in]
        n578 = Unbundle By Name(w1457) -> ("ROI Type"=w1458:u32)
        n579 = Not Equal To 0?(x=w1458) -> (x != 0?=w1459:bool)
        n580 = And(x="Save current ROI", y=w1459) -> (x .and. y?=w1462:bool)
        n581 = case shown="True" w1462 {
          tunnel: w1461 -> [_ w1473]
          frame False {
          }
          frame True {
            n582 = control-ref of="This VI"() -> (w1477:refnum<vi>)
            n583 = property class="VI"(reference=w1477) -> ("Path"=w1478:path)  [unwired: 1 in, 2 out]
            n584 = call "IMAQ Create"("Image Name"="untitled") -> ("New Image"=w1474:T2)  [unwired: 4 in, 1 out]
            n585 = call "IMAQ ROIToMask 2"("ROI Descriptor"=w1473, "Image"=w1474) -> ("Image Out"=w1476:T2)  [unwired: 7 in, 2 out]
            n586 = Strip Path(path=w1478) -> (stripped path=w1479:path)  [unwired: 1 out]
            n587 = Build Path(base path=w1479, name or relative path="Saved ROI") -> (appended path=w1472:path)
            n588 = call <vilib>:"Check if File or Folder Exists.vi"("path"=w1472) -> ("file or folder exists?"=w1471:bool, "dup path"=w1470:path)  [unwired: 8 in, 1 out]
            n589 = case shown="True" w1471 {
              tunnel: w1470 -> [w1482 w1483]
              tunnel: [w1481 w1483] -> w1469
              frame False {
                n590 = Create Folder(path (use dialog)=w1482) -> (created path=w1481:path)  [unwired: 2 in, 2 out]
              }
              frame True {
              }
            }
            n591 = Get Date/Time In Seconds() -> (seconds since 1Jan1904=w1466:timestamp)
            n592 = Format Date/Time String(time format string (%c)="%d%m%y %I-%M %p ", seconds (now)=w1466) -> (date/time string=w1465:string)  [unwired: 1 in]
            n593 = Concatenate Strings(w1465, " - saved ROI.tiff" ("string")) -> (w1463:string)
            n594 = Build Path(base path=w1469, name or relative path=w1463) -> (appended path=w1468:path)
            n595 = call-poly "IMAQ Write File 2"("File Path"=w1468, "Image"=w1476) -> ()  [unwired: 8 in, 2 out]
          }
        }
      }
      event "Load ROI": Value Change {
        n596 = event-data() -> ()  [unwired: 1 in, 6 out]
        n597 = case shown="True" "Load ROI" {
          frame False {
          }
          frame True {
            n598 = call "File Dialog"("prompt"="Select an ROI file..." ("pattern label"), "pattern (all files)"="*.jpg;*.bmp;*.jpeg;*.tif;*.tiff;*.png", "pattern label"="ROI files") -> ("selected path"=w1485:path, "cancelled"=w1486:bool)  [unwired: 9 in, 2 out]